vi "Controle_Manip_Main_GUI_Backup2.vi"() -> ()   [LabVIEW 2019] (continued)
                      }
                    }
                    n2428 = local read "ourDLL"() -> (w2916:path)
                    n2429 = call "ANC_MoveAbs.vi"("Att DeviceHandle"=w2915, "ourDLL"=w2916, "axis"=w2918, "Target pos"=w2919, "Att Error"=w2914) -> ("deviceHandle out"=w2913:u64, "Out Position [µm | m°]"=→"Out Position [µm | m°]":dbl, "error out"=w2912:errorcluster)  [unwired: 1 in]
                    n2430 = local write "Att DeviceHandle"(w2913) -> ()
                    n2431 = local write "Att Error"(w2912) -> ()
                  }
                }
              }
              frame #1 {
                n2432 = property on="Att Read Pos" class="Bool (strict)"("Val(Sgnl)"=TRUE ("Value (Signaling)")) -> ()  [unwired: 2 in, 2 out]
              }
            }
          }
          event "Att Read Pos": Value Change {
            n2433 = event-data() -> ()  [unwired: 1 in, 6 out]
            n2434 = flat-sequence {
              frame #0 {
                w2929 = u8 2 items=["1", "2", "3"] ("axis")
                w2930 = u8 1 items=["1", "2", "3"] ("axis")
                w2931 = u8 0 items=["1", "2", "3"] ("axis")
                n2435 = local read "Att DeviceHandle"() -> (w2943:u64)
                n2436 = local read "Att Error"() -> (w2942:errorcluster)
                n2437 = local read "ourDLL"() -> (w2937:path)
                n2438 = call "ANC350v4_GetPosition.vi"("deviceHandle"=w2943, "Path to *.DLL"=w2937, "axis"=w2931, "error in"=w2942) -> ("deviceHandle"=w2941:u64, "Position [µm | m°]"=w2936:dbl, "error ANC350v4_getPosition"=w2940:errorcluster)  [unwired: 8 in, 1 out]
                n2439 = call "ANC350v4_GetPosition.vi"("deviceHandle"=w2941, "Path to *.DLL"=w2937, "axis"=w2930, "error in"=w2940) -> ("deviceHandle"=w2939:u64, "Position [µm | m°]"=w2935:dbl, "error ANC350v4_getPosition"=w2938:errorcluster)  [unwired: 8 in, 1 out]
                n2440 = local write "Att Pos Y"(w2936) -> ()
                n2441 = local write "Att Pos X"(w2935) -> ()
                n2442 = call "ANC350v4_GetPosition.vi"("deviceHandle"=w2939, "Path to *.DLL"=w2937, "axis"=w2929, "error in"=w2938) -> ("deviceHandle"=w2933:u64, "Position [µm | m°]"=w2934:dbl, "error ANC350v4_getPosition"=w2932:errorcluster)  [unwired: 8 in, 1 out]
                n2443 = local write "Att DeviceHandle"(w2933) -> ()
                n2444 = local write "Att Pos Z"(w2934) -> ()
                n2445 = local write "Att Error"(w2932) -> ()
              }
              frame #1 {
                n2446 = local write "Att Read Pos"(FALSE ("Att Read Pos")) -> ()
              }
            }
          }
          event "Att Track Target": Value Change {
            n2447 = event-data() -> ("NewVal"=w2945:bool)  [unwired: 1 in, 5 out]
            n2448 = case shown="False" w2945 {
              frame False {
                w2956 = u8 2 items=["1", "2", "3"] ("axis")
                w2957 = u8 1 items=["1", "2", "3"] ("axis")
                w2962 = u8 0 items=["1", "2", "3"] ("axis")
                n2449 = local read "Att DeviceHandle"() -> (w2950:u64)
                n2450 = local read "Att Error"() -> (w2949:errorcluster)
                n2451 = local read "ourDLL"() -> (w2946:path)
                n2452 = call "ANC350v4_StartAutoMove.vi"("deviceHandle"=w2950, "Path to *.DLL"=w2946, "axis"=w2962, "Enable | Disable"=FALSE, "Relative | Absolute"=TRUE, "error in"=w2949) -> ("deviceHandle out"=w2961:u64, "error ANC350v4_StartAutoMove"=w2960:errorcluster)  [unwired: 7 in, 1 out]
                n2453 = call "ANC350v4_StartAutoMove.vi"("deviceHandle"=w2961, "Path to *.DLL"=w2946, "axis"=w2957, "Enable | Disable"=FALSE, "Relative | Absolute"=TRUE, "error in"=w2960) -> ("deviceHandle out"=w2959:u64, "error ANC350v4_StartAutoMove"=w2958:errorcluster)  [unwired: 7 in, 1 out]
                n2454 = call "ANC350v4_StartAutoMove.vi"("deviceHandle"=w2959, "Path to *.DLL"=w2946, "axis"=w2956, "Enable | Disable"=FALSE, "Relative | Absolute"=TRUE, "error in"=w2958) -> ("deviceHandle out"=w2948:u64, "error ANC350v4_StartAutoMove"=w2947:errorcluster)  [unwired: 7 in, 1 out]
                n2455 = local write "Att DeviceHandle"(w2948) -> ()
                n2456 = local write "Att Error"(w2947) -> ()
              }
              frame True {
              }
            }
          }
          event "Att Up", "Att Down", "Att Left", "Att Right", "Att Backward", "Att Forward": Value Change {
            n2457 = event-data() -> ("CtlRef"=w2965:refnum<vi>, "NewVal"=w2966:bool)  [unwired: 1 in, 4 out]
            n2458 = local read "Voltage Output?"() -> (w2964:bool)
            n2459 = case shown="True" w2964 {
              tunnel: w2966 -> [_ w2969]
              tunnel: w2965 -> [_ w2968]
              frame False {
              }
              frame True {
                n2460 = local read "Att DeviceHandle"() -> (w2974:u64)
                n2461 = local read "ourDLL"() -> (w2971:path)
                n2462 = local read "Att Error"() -> (w2973:errorcluster)
                n2463 = local read "Att Mode"() -> (w2975:enum16{"Single Step", "Continuous", "Automatic"})
                n2464 = property class="Bool (strict)"(reference=w2968) -> ("Label.Text"=w2972:string)  [unwired: 1 in, 2 out]
                n2465 = case shown="\"Automatic\"" w2975 {
                  tunnel: w2974 -> [w2979 w3017 w3064]
                  tunnel: w2973 -> [w2980 w3018 w3063]
                  tunnel: w2972 -> [w2978 w3021 w3045]
                  tunnel: w2971 -> [w2984 w3014 w3056]
                  tunnel: [w2983 w3024 w3068] -> w2970
                  tunnel: [w2982 w3023 w3067] -> w2967
                  tunnel: w2969 -> [_ w3020 _]
                  tunnel: w2968 -> [_ _ w3048]
                  frame "Single Step", Default {
                    n2466 = case shown="\"Att Up\"" w2978 {
                      tunnel: [FALSE ("direction [t=bwd | f=fwd]") TRUE FALSE ("direction [t=bwd | f=fwd]") TRUE ("direction [t=bwd | f=fwd]") FALSE ("direction [t=bwd | f=fwd]") TRUE ("direction [t=bwd | f=fwd]")] -> w2987
                      tunnel: [w3000 w3002 w3005 w3006 w3009 w3010] -> w2981
                      frame "Att Forward" {
                        w3000 = u8 2 items=["1", "2", "3"] ("axis")
                      }
                      frame "Att Backward" {
                        w3002 = u8 2 items=["1", "2", "3"] ("axis")
                      }
                      frame "Att Up" {
                        w3005 = u8 0 items=["1", "2", "3"] ("axis")
                      }
                      frame "Att Down", Default {
                        w3006 = u8 0 items=["1", "2", "3"] ("axis")
                      }
                      frame "Att Left" {
                        w3009 = u8 1 items=["1", "2", "3"] ("axis")
                      }
                      frame "Att Right" {
                        w3010 = u8 1 items=["1", "2", "3"] ("axis")
                      }
                    }
                    n2467 = call "ANC350v4_SingleStep.vi"("deviceHandle"=w2979, "Path to *.DLL"=w2984, "axis"=w2981, "direction [t=bwd | f=fwd]"=w2987, "error in"=w2980) -> ("deviceHandle"=w2985:u64, "error ANC350v4_singleStep"=w2986:errorcluster)  [unwired: 8 in, 1 out]
                    n2468 = call "ANC350v4_GetPosition.vi"("deviceHandle"=w2985, "Path to *.DLL"=w2984, "axis"=w2981, "error in"=w2986) -> ("deviceHandle"=w2983:u64, "Position [µm | m°]"=w2977:dbl, "error ANC350v4_getPosition"=w2982:errorcluster)  [unwired: 8 in, 1 out]
                    n2469 = case shown="\"Att Backward\"" w2978 {
                      tunnel: w2977 -> [w2989 w2991 w2993 w2995 w2997 _ w2999]
                      tunnel: FALSE -> [w2988 w2990 w2992 w2994 w2996 _ w2998]
                      frame "Att Right" {
                        n2470 = local write "Att Right"(w2988) -> ()
                        n2471 = local write "Att Pos X"(w2989) -> ()
                      }
                      frame "Att Left" {
                        n2472 = local write "Att Left"(w2990) -> ()
                        n2473 = local write "Att Pos X"(w2991) -> ()
                      }
                      frame "Att Up" {
                        n2474 = local write "Att Up"(w2992) -> ()
                        n2475 = local write "Att Pos Y"(w2993) -> ()
                      }
                      frame "Att Down" {
                        n2476 = local write "Att Down"(w2994) -> ()
                        n2477 = local write "Att Pos Y"(w2995) -> ()
                      }
                      frame "Att Forward" {
                        n2478 = local write "Att Forward"(w2996) -> ()
                        n2479 = local write "Att Pos Z"(w2997) -> ()
                      }
                      frame "False", Default {
                      }
                      frame "Att Backward" {
                        n2480 = local write "Att Backward"(w2998) -> ()
                        n2481 = local write "Att Pos Z"(w2999) -> ()
                      }
                    }
                  }
                  frame "Continuous" {
                    n2482 = case shown="False" w3020 {
                      tunnel: [FALSE TRUE] -> w3015
                      frame False {
                      }
                      frame True {
                      }
                    }
                    n2483 = case shown="\"Att Left\"" w3021 {
                      tunnel: [FALSE ("direction [t=bwd | f=fwd]") TRUE FALSE ("direction [t=bwd | f=fwd]") TRUE ("direction [t=bwd | f=fwd]") FALSE ("direction [t=bwd | f=fwd]") TRUE ("direction [t=bwd | f=fwd]")] -> w3019
                      tunnel: [w3033 w3035 w3038 w3039 w3042 w3043] -> w3016
                      frame "Att Forward" {
                        w3033 = u8 2 items=["1", "2", "3"] ("axis")
                      }
                      frame "Att Backward" {
                        w3035 = u8 2 items=["1", "2", "3"] ("axis")
                      }
                      frame "Att Up" {
                        w3038 = u8 0 items=["1", "2", "3"] ("axis")
                      }
                      frame "Att Down", Default {
                        w3039 = u8 0 items=["1", "2", "3"] ("axis")
                      }
                      frame "Att Left" {
                        w3042 = u8 1 items=["1", "2", "3"] ("axis")
                      }
                      frame "Att Right" {
                        w3043 = u8 1 items=["1", "2", "3"] ("axis")
                      }
                    }
                    n2484 = call "ANC350v4_StartContinousMove.vi"("deviceHandle"=w3017, "Path to *.DLL"=w3014, "axis"=w3016, "start | stop"=w3015, "direction [t=bwd | f=fwd]"=w3019, "error in"=w3018) -> ("deviceHandle"=w3012:u64, "error ANC350v4_startContinousMove"=w3013:errorcluster)  [unwired: 7 in, 1 out]
                    n2485 = call "ANC350v4_GetPosition.vi"("deviceHandle"=w3012, "Path to *.DLL"=w3014, "axis"=w3016, "error in"=w3013) -> ("deviceHandle"=w3024:u64, "Position [µm | m°]"=w3022:dbl, "error ANC350v4_getPosition"=w3023:errorcluster)  [unwired: 8 in, 1 out]
                    n2486 = case shown="\"Att Right\"" w3021 {
                      tunnel: w3022 -> [_ w3027 w3028 w3029 w3030 w3031 w3032]
                      frame "False", Default {
                      }
                      frame "Att Right" {
                        n2487 = local write "Att Pos X"(w3027) -> ()
                      }
                      frame "Att Left" {
                        n2488 = local write "Att Pos X"(w3028) -> ()
                      }
                      frame "Att Up" {
                        n2489 = local write "Att Pos Y"(w3029) -> ()
                      }
                      frame "Att Down" {
                        n2490 = local write "Att Pos Y"(w3030) -> ()
                      }
                      frame "Att Forward" {
                        n2491 = local write "Att Pos Z"(w3031) -> ()
                      }
                      frame "Att Backward" {
                        n2492 = local write "Att Pos Z"(w3032) -> ()
                      }
                    }
                  }
                  frame "Automatic" {
                    n2493 = local read "Att AutoStep"() -> (w3046:dbl)
                    n2494 = case shown="\"Att Right\"" w3045 {
                      tunnel: [w3110 w3113 w3115 w3118 w3120 w3123] -> w3057
                      tunnel: [w3109 w3111 w3114 w3117 w3119 w3121] -> w3047
                      tunnel: w3046 -> [w3109 w3112 w3114 w3116 w3119 w3122]
                      frame "Att Forward" {
                        w3110 = u8 2 items=["1", "2", "3"] ("axis")
                      }
                      frame "Att Backward" {
                        w3113 = u8 2 items=["1", "2", "3"] ("axis")
                        n2495 = Negate(x=w3112) -> (-x=w3111:dbl)
                      }
                      frame "Att Up" {
                        w3115 = u8 0 items=["1", "2", "3"] ("axis")
                      }
                      frame "Att Down", Default {
                        w3118 = u8 0 items=["1", "2", "3"] ("axis")
                        n2496 = Negate(x=w3116) -> (-x=w3117:dbl)
                      }
                      frame "Att Left" {
                        w3120 = u8 1 items=["1", "2", "3"] ("axis")
                      }
                      frame "Att Right" {
                        w3123 = u8 1 items=["1", "2", "3"] ("axis")
                        n2497 = Negate(x=w3122) -> (-x=w3121:dbl)
                      }
                    }
                    n2498 = call "ANC350v4_SetTarget.vi"("deviceHandle"=w3064, "Path to *.DLL"=w3056, "axis"=w3057, "Target [µm | m°]"=w3047, "error in"=w3063) -> ("deviceHandle"=w3065:u64, "error ANC350v4_setTarget"=w3062:errorcluster)  [unwired: 8 in, 1 out]
                    n2499 = call "ANC350v4_StartAutoMove.vi"("deviceHandle"=w3065, "Path to *.DLL"=w3056, "axis"=w3057, "Enable | Disable"=TRUE, "Relative | Absolute"=TRUE, "error in"=w3062) -> ("deviceHandle out"=w3058:u64, "error ANC350v4_StartAutoMove"=w3059:errorcluster)  [unwired: 7 in, 1 out]
                    n2500 = while {
                      tunnel: w3059 -> [w3102]
                      tunnel: w3058 -> [w3101]
                      tunnel: w3057 -> [w3091]
                      tunnel: w3056 -> [w3090]
                      tunnel: [w3094] -> w3052
                      tunnel: [w3093] -> w3051
                      tunnel: [w3090] -> w3050
                      tunnel: [w3091] -> w3049
                      tunnel: w3045 -> [w3089]
                      stop <- w3098 stop-if-true
                      n2501 = call "ANC350v4_GetAxisStatus.vi"("deviceHandle"=w3101, "Path to *.DLL"=w3090, "axis"=w3091, "error in"=w3102) -> ("deviceHandle"=w3095:u64, "Target"=w3099:bool, "error ANC350v4_getAxisStatus"=w3092:errorcluster)  [unwired: 6 in, 3 out]
                      n2502 = Wait (ms)(milliseconds to wait=u32 250) -> ()  [unwired: 1 out]
                      n2503 = call "ANC350v4_GetPosition.vi"("deviceHandle"=w3095, "Path to *.DLL"=w3090, "axis"=w3091, "error in"=w3092) -> ("deviceHandle"=w3094:u64, "Position [µm | m°]"=w3096:dbl, "error ANC350v4_getPosition"=w3093:errorcluster)  [unwired: 8 in, 1 out]
                      n2504 = case shown="\"Att Down\"" w3089 {
                        tunnel: w3096 -> [_ w3103 w3104 w3105 w3106 w3107 w3108]
                        frame "False", Default {
                        }
                        frame "Att Right" {
                          n2505 = local write "Att Pos X"(w3103) -> ()
                        }
                        frame "Att Left" {
                          n2506 = local write "Att Pos X"(w3104) -> ()
                        }
                        frame "Att Up" {
                          n2507 = local write "Att Pos Y"(w3105) -> ()
                        }
                        frame "Att Down" {
                          n2508 = local write "Att Pos Y"(w3106) -> ()
                        }
                        frame "Att Forward" {
                          n2509 = local write "Att Pos Z"(w3107) -> ()
                        }
                        frame "Att Backward" {
                          n2510 = local write "Att Pos Z"(w3108) -> ()
                        }
                      }
                      n2511 = Or(x=w3099, y="Att Stop Target Wait") -> (x .or. y?=w3098:bool)
                    }
                    n2512 = local read "Att Track Target"() -> (w3053:bool)
                    n2513 = case shown="False" w3053 {
                      tunnel: w3052 -> [w3085 w3088]
                      tunnel: w3051 -> [w3084 w3087]
                      tunnel: [w3082 w3088] -> w3055
                      tunnel: [w3083 w3087] -> w3054
                      tunnel: w3050 -> [w3086 _]
                      tunnel: w3049 -> [w3081 _]
                      frame False {
                        n2514 = call "ANC350v4_StartAutoMove.vi"("deviceHandle"=w3085, "Path to *.DLL"=w3086, "axis"=w3081, "Enable | Disable"=FALSE, "Relative | Absolute"=TRUE, "error in"=w3084) -> ("deviceHandle out"=w3082:u64, "error ANC350v4_StartAutoMove"=w3083:errorcluster)  [unwired: 7 in, 1 out]
                      }
                      frame True {
                      }
                    }
                    n2515 = call "ANC350v4_GetPosition.vi"("deviceHandle"=w3055, "Path to *.DLL"=w3056, "axis"=w3057, "error in"=w3054) -> ("deviceHandle"=w3068:u64, "Position [µm | m°]"=w3066:dbl, "error ANC350v4_getPosition"=w3067:errorcluster)  [unwired: 8 in, 1 out]
                    n2516 = stacked-sequence {
                      tunnel: w3066 -> [w3070 _]
                      tunnel: w3045 -> [w3069 _]
                      tunnel: w3048 -> [_ w3077]
                      frame #0 {
                        n2517 = case shown="\"Att Right\"" w3069 {
                          tunnel: w3070 -> [_ w3071 w3072 w3073 w3074 w3075 w3076]
                          frame "False", Default {
                          }
                          frame "Att Right" {
                            n2518 = local write "Att Pos X"(w3071) -> ()
                          }
                          frame "Att Left" {
                            n2519 = local write "Att Pos X"(w3072) -> ()
                          }
                          frame "Att Up" {
                            n2520 = local write "Att Pos Y"(w3073) -> ()
                          }
                          frame "Att Down" {
                            n2521 = local write "Att Pos Y"(w3074) -> ()
                          }
                          frame "Att Forward" {
                            n2522 = local write "Att Pos Z"(w3075) -> ()
                          }
                          frame "Att Backward" {
                            n2523 = local write "Att Pos Z"(w3076) -> ()
                          }
                        }
                      }
                      frame #1 {
                        n2524 = property class="Bool (strict)"(reference=w3077, "Value"=FALSE) -> ()  [unwired: 1 in, 2 out]
                      }
                    }
                  }
                }
                n2525 = local write "Att DeviceHandle"(w2970) -> ()
                n2526 = local write "Att Error"(w2967) -> ()
              }
            }
          }
          event "Att Wobble Get Pos 1", "Att Wobble Get Pos 2", "Att Wobble": Mouse Down {
            n2527 = event-data() -> ("CtlRef"=w3125:refnum<vi>)  [unwired: 1 in, 7 out]
            n2528 = property class="Bool (strict)"(reference=w3125) -> ("Label.Text"=w3124:string)  [unwired: 1 in, 2 out]
            n2529 = case shown="\"Att Wobble\"" w3124 {
              frame "Att Wobble" {
                n2530 = stacked-sequence {
                  frame #0 {
                    n2531 = local read "Att DeviceHandle"() -> (w3132:u64)
                    n2532 = local read "Att Wobble Start"() -> (w3134:dbl)
                    n2533 = local read "Att Wobble End"() -> (w3133:dbl)
                    n2534 = control-ref of="Att Wobble Stop2"() -> (w3127:refnum<vi>)
                    n2535 = local read "Att Error"() -> (w3131:errorcluster)
                    n2536 = local read "ourDLL"() -> (w3130:path)
                    n2537 = control-ref of="Att Pos Z"() -> (w3126:refnum<vi>)
                    n2538 = call "Att_Wobble.vi"("Att Pos Z"=w3126, "Att Wobble End"=w3133, "Att Wobble Start"=w3134, "Att Error"=w3131, "ourDLL"=w3130, "Att Wobble Stop2 2"=w3127, "Att DeviceHandle"=w3132) -> ("Att Error out"=w3128:errorcluster, "Att DeviceHandle out"=w3129:u64)  [unwired: 1 in]
                    n2539 = local write "Att DeviceHandle"(w3129) -> ()
                    n2540 = local write "Att Error"(w3128) -> ()
                  }
                  frame #1 {
                    w3135 = FALSE ("Att Wobble")
                    n2541 = local write "Att Wobble Stop2"(w3135) -> ()
                    n2542 = local write "Att Wobble"(w3135) -> ()
                  }
                }
              }
              frame "False", Default {
              }
              frame "Att Wobble Get Pos 1" {
                n2543 = property on="Att Pos Z" class="DigNum (strict)"() -> ("Value"=w3136:dbl)  [unwired: 2 in, 2 out]
                n2544 = local write "Att Wobble Start"(w3136) -> ()
              }
              frame "Att Wobble Get Pos 2" {
                n2545 = property on="Att Pos Z" class="DigNum (strict)"() -> ("Value"=w3137:dbl)  [unwired: 2 in, 2 out]
                n2546 = local write "Att Wobble End"(w3137) -> ()
              }
            }
          }
          event "Auto< ?": Value Change {
            n2547 = event-data() -> ("NewVal"=w3138:bool)  [unwired: 1 in, 5 out]
            n2548 = case shown="True" w3138 {
              frame False {
                w3139 = TRUE ("Visible")
                n2549 = property on="Save Spectrum N" class="Bool (strict)"("Visible"=w3139) -> ()  [unwired: 2 in, 2 out]
                n2550 = property on="Save XY Map" class="Bool (strict)"("Visible"=w3139) -> ()  [unwired: 2 in, 2 out]
                n2551 = property on="Save Spectrum" class="Bool (strict)"("Visible"=w3139) -> ()  [unwired: 2 in, 2 out]
                n2552 = property on="Save PLE" class="Bool (strict)"("Visible"=w3139) -> ()  [unwired: 2 in, 2 out]
                n2553 = property on="Save fPow" class="Bool (strict)"("Visible"=w3139) -> ()  [unwired: 2 in, 2 out]
                n2554 = property on="Save Custom Diode Spectrum" class="Bool (strict)"("Visible"=w3139) -> ()  [unwired: 2 in, 2 out]
                n2555 = property on="Save Michelson" class="Bool (strict)"("Visible"=w3139) -> ()  [unwired: 2 in, 2 out]
                n2556 = property on="Save Polarisation" class="Bool (strict)"("Visible"=w3139) -> ()  [unwired: 2 in, 2 out]
                n2557 = property on="Save Contrast" class="Bool (strict)"("Visible"=w3139) -> ()  [unwired: 2 in, 2 out]
              }
              frame True {
                w3140 = FALSE ("Visible")
                n2558 = property on="Save Spectrum N" class="Bool (strict)"("Visible"=w3140) -> ()  [unwired: 2 in, 2 out]
                n2559 = property on="Save XY Map" class="Bool (strict)"("Visible"=w3140) -> ()  [unwired: 2 in, 2 out]
                n2560 = property on="Save Spectrum" class="Bool (strict)"("Visible"=w3140) -> ()  [unwired: 2 in, 2 out]
                n2561 = property on="Save PLE" class="Bool (strict)"("Visible"=w3140) -> ()  [unwired: 2 in, 2 out]
                n2562 = property on="Save fPow" class="Bool (strict)"("Visible"=w3140) -> ()  [unwired: 2 in, 2 out]
                n2563 = property on="Save Polarisation" class="Bool (strict)"("Visible"=w3140) -> ()  [unwired: 2 in, 2 out]
                n2564 = property on="Save Michelson" class="Bool (strict)"("Visible"=w3140) -> ()  [unwired: 2 in, 2 out]
                n2565 = property on="Save Contrast" class="Bool (strict)"("Visible"=w3140) -> ()  [unwired: 2 in, 2 out]
                n2566 = property on="Save Custom Diode Spectrum" class="Bool (strict)"("Visible"=w3140) -> ()  [unwired: 2 in, 2 out]
              }
            }
          }
          event "Background substract": Value Change {
            n2567 = event-data() -> ("NewVal"=w3141:enum16{"None", "Shutter"})  [unwired: 1 in, 5 out]
            n2568 = case shown="\"Shutter\"" w3141 {
              frame "None", Default {
              }
              frame "Shutter" {
                n2569 = stacked-sequence {
                  tunnel: [_ _ w3191] -> w3142
                  frame #0 {
                    n2570 = local read "Log file"() -> (w3176:string)
                    n2571 = property on="CCD 1D Spectrum Main" class="XYGraph (strict)"("YScale.Offset"=0.0 ("Y Scale.Offset and Multiplier:Offset")) -> ()  [unwired: 2 in, 2 out]
                    n2572 = call "Write2LogFile.vi"("Add to log file"="Acquiring background", "Log file before"=w3176, "Checkbox"=FALSE) -> ("Log file after"=w3175:string)
                    n2573 = local write "Log file"(w3175) -> ()
                  }
                  frame #1 {
                    # "make sure shutter is closed"
                    n2574 = local read "KCube Shutter On?"() -> (w3177:bool)
                    n2575 = control-ref of="Shutter Ctrls"() -> (w3181:refnum<vi>)
                    n2576 = property class="Ring (strict)"(reference=w3181) -> ("Value"=w3180:u16)  [unwired: 1 in, 2 out]
                    n2577 = control-ref of="KCube Shutter Device Reference"() -> (w3182:refnum<vi>)
                    n2578 = Equal?(x=w3180, y=u16 0) -> (x = y?=w3178:bool)
                    n2579 = case shown="False" w3178 {
                      tunnel: w3182 -> [w3185 _]
                      tunnel: w3181 -> [w3184 _]
                      tunnel: w3177 -> [w3183 _]
                      frame False {
                        n2580 = call "Shutter.vi"("KCube Shutter Device Reference 2"=w3185, "Shutter Ctrls 2"=w3184, "Shutter on?"=w3183) -> ()
                      }
                      frame True {
                      }
                    }
                  }
                  frame #2 {
                    # "acquire"
                    n2581 = local read "LightField Automation error out"() -> (w3189:errorcluster)
                    n2582 = local read "LightField Automation out"() -> (w3190:refnum<class "LightField Automation.lvclass">)
                    n2583 = local read "Accumulations"() -> (w3186:dbl)
                    n2584 = call "LFA_Capture.vi"("error in (no error)"=w3189, "Frames"=w3186, "LightField Automation in"=w3190) -> ("error out"=w3188:errorcluster, "Data"=w3191:T26, "LightField Automation out"=w3187:refnum<class "LightField Automation.lvclass">)  [unwired: 6 in]
                    n2585 = local write "LightField Automation error out"(w3188) -> ()
                    n2586 = local write "LightField Automation out"(w3187) -> ()
                  }
                }
                n2587 = local read "Acq Mode"() -> (w3143:T3)
                n2588 = case shown="\"Spectrum\", Default" w3143 {
                  selector: w3143 -> [w3144 w3162]
                  tunnel: w3142 -> [w3145 w3163]
                  frame "Spectrum", Default {
                    n2589 = stacked-sequence {
                      tunnel: w3145 -> [_ w3156 _ _]
                      tunnel: w3144 -> [_ w3154 _ _]
                      frame #0 {
                        n2590 = property on="CCD 2D Image Main" class="IntGraph (strict)"("Visible"=FALSE) -> ()  [unwired: 2 in, 2 out]
                        n2591 = property on="CCD 1D Spectrum Main" class="XYGraph (strict)"("Visible"=TRUE) -> ()  [unwired: 2 in, 2 out]
                      }
                      frame #1 {
                        n2592 = local read "CCD ROI"() -> (w3149:T20)
                        n2593 = local read "Wavelength calibration"() -> (w3153:dbl[])
                        n2594 = Divide(x=1239.842, y=w3153) -> (x/y=w3151:dbl[])
                        n2595 = call "PrepareData4Graph.vi"("Wavelength nm"=w3151, "DataLF"=w3156, "CCD ROI"=w3149, "AcqMode"=w3154, "Data type"=T30."Spectre") -> ("Spectrum"=w3155:cluster{"Array 2":dbl[], "Array":dbl[]}, "PLInt out"=w3148:dbl[])  [unwired: 2 in, 2 out]
                        n2596 = local write "CCD 1D Spectrum Main"(w3155) -> ()
                        n2597 = local write "BackgroundSpec"(w3148) -> ()
                      }
                      frame #2 {
                        n2598 = local read "BackgroundSpec"() -> (w3157:dbl[])
                        n2599 = call-poly <vilib>:"Mean.vi"("X"=w3157) -> ("mean"=w3159:dbl)  [unwired: 1 out]
                        n2600 = Negate(x=w3159) -> (-x=w3158:dbl)
                        n2601 = property on="CCD 1D Spectrum Main" class="XYGraph (strict)"("YScale.Offset"=w3158) -> ()  [unwired: 2 in, 2 out]
                      }
                      frame #3 {
                        n2602 = local write "Background taken?"(TRUE ("Background taken?")) -> ()
                        n2603 = property on="Background substract" class="Enum (strict)"("Value"=enum16{"None", "Shutter"}."None" ("Background substract")) -> ()  [unwired: 2 in, 2 out]
                      }
                    }
                  }
                  frame "Image" {
                    n2604 = stacked-sequence {
                      tunnel: w3163 -> [_ w3171]
                      tunnel: w3162 -> [_ w3169]
                      frame #0 {
                        n2605 = property on="CCD 1D Spectrum Main" class="XYGraph (strict)"("Visible"=FALSE) -> ()  [unwired: 2 in, 2 out]
                        n2606 = property on="CCD 2D Image Main" class="IntGraph (strict)"("Visible"=TRUE) -> ()  [unwired: 2 in, 2 out]
                      }
                      frame #1 {
                        n2607 = local read "Wavelength calibration"() -> (w3170:dbl[])
                        n2608 = local read "CCD ROI"() -> (w3166:T20)
                        n2609 = call "PrepareData4Graph.vi"("Wavelength nm"=w3170, "DataLF"=w3171, "CCD ROI"=w3166, "AcqMode"=w3169, "Data type"=T30."Spectre") -> ("Intensity Graph"=w3168:dbl[][])  [unwired: 2 in, 3 out]
                        n2610 = local write "CCD 2D Image Main"(w3168) -> ()
                      }
                    }
                  }
                }
              }
            }
          }
          event "CCD 1D Spectrum Main  Cursor2WL 1 Mono 1", "CCD 1D Spectrum Main  Cursor2WL 2 Mono 1", "CCD 1D Spectrum Main  Cursor2WL 1 Mono 2", "CCD 1D Spectrum Main  Cursor2WL 2 Mono 2": Mouse Down {
            n2611 = event-data() -> ("CtlRef"=w3193:refnum<vi>)  [unwired: 1 in, 7 out]
            n2612 = property class="Bool (strict)"(reference=w3193) -> ("Label.Text"=w3192:string)  [unwired: 1 in, 2 out]
            n2613 = case shown="Default" w3192 {
              frame "CCD 1D Spectrum Main  Cursor2WL 1 Mono 1" {
                n2614 = local read "CCD 1D Spectrum Main Cursor 1 nm"() -> (w3194:dbl)
                n2615 = property on="Center Wavelength (nm)" class="DigNum (strict)"("Val(Sgnl)"=w3194) -> ()  [unwired: 2 in, 2 out]
              }
              frame "CCD 1D Spectrum Main  Cursor2WL 1 Mono 2" {
                n2616 = local read "CCD 1D Spectrum Main Cursor 1 nm"() -> (w3195:dbl)
                n2617 = property on="Mono2 Wavelength (nm)" class="DigNum (strict)"("Val(Sgnl)"=w3195) -> ()  [unwired: 2 in, 2 out]
              }
              frame "CCD 1D Spectrum Main  Cursor2WL 2 Mono 2" {
                n2618 = local read "CCD 1D Spectrum Main Cursor 2 nm"() -> (w3196:dbl)
                n2619 = property on="Mono2 Wavelength (nm)" class="DigNum (strict)"("Val(Sgnl)"=w3196) -> ()  [unwired: 2 in, 2 out]
              }
              frame "CCD 1D Spectrum Main  Cursor2WL 2 Mono 1" {
                n2620 = local read "CCD 1D Spectrum Main Cursor 2 nm"() -> (w3197:dbl)
                n2621 = property on="Center Wavelength (nm)" class="DigNum (strict)"("Val(Sgnl)"=w3197) -> ()  [unwired: 2 in, 2 out]
              }
              frame Default {
              }
            }
          }
          event "CCD 1D Spectrum Main", "Contrast Oscillations", "Contrast 1D Spectrum": Cursor Release {
            n2622 = event-data() -> ("CtlRef"=w3201:refnum<vi>, "CursRef"=w3199:refnum<vi>)  [unwired: 1 in, 7 out]
            n2623 = property class="XYGraph (strict)"(reference=w3201) -> ("Label.Text"=w3200:string)  [unwired: 1 in, 2 out]
            n2624 = property class="Curs"(reference=w3199) -> ("Cursor Name"=w3198:string)  [unwired: 1 in, 2 out]
            n2625 = case shown="\"Contrast 1D Spectrum\"" w3200 {
              tunnel: w3198 -> [w3202 _ _ _]
              frame "Contrast Oscillations" {
                n2626 = case shown="\"ContPos\"" w3202 {
                  frame "False", Default {
                  }
                  frame "ContPos" {
                    n2627 = local read "Cursor controls"() -> (w3203:bool)
                    n2628 = case shown="True" w3203 {
                      frame False {
                      }
                      frame True {
                        n2629 = property on="Contrast Oscillations" class="XYGraph (strict)"("Active Cursor"=u32 2) -> ("Cursor.Cursor X"=w3204:dbl)  [unwired: 2 in, 2 out]
                        n2630 = Number To Decimal String(number=w3204) -> (decimal integer string=w3206:string)  [unwired: 1 in]
                        n2631 = property on="Contrast 1D Spectrum from Cursors" class="XYGraph (strict)"("Caption.Text"=w3206) -> ()  [unwired: 2 in, 2 out]
                      }
                    }
                  }
                  frame "ContInt1" {
                    n2632 = property on="Contrast Oscillations" class="XYGraph (strict)"("Active Cursor"=u32 0, "Active Cursor"=u32 1) -> ("Cursor.Cursor Y"=w3209:dbl, "Cursor.Cursor Y"=w3208:dbl)  [unwired: 2 in, 2 out]
                    n2633 = call "Contrast.vi"("Y2"=w3208, "Y1"=w3209) -> ("(max(Y1,Y2) - min(Y1,Y2)) / (Y1 + Y2)"=w3207:dbl)
                    n2634 = local write "Contrast"(w3207) -> ()
                  }
                  frame "ContInt2" {
                    n2635 = property on="Contrast Oscillations" class="XYGraph (strict)"("Active Cursor"=u32 0, "Active Cursor"=u32 1) -> ("Cursor.Cursor Y"=w3214:dbl, "Cursor.Cursor Y"=w3213:dbl)  [unwired: 2 in, 2 out]
                    n2636 = call "Contrast.vi"("Y2"=w3213, "Y1"=w3214) -> ("(max(Y1,Y2) - min(Y1,Y2)) / (Y1 + Y2)"=w3212:dbl)
                    n2637 = local write "Contrast"(w3212) -> ()
                  }
                }
              }
              frame "Contrast 1D Spectrum" {
                n2638 = case shown="True" "Cursor controls" {
                  frame False {
                  }
                  frame True {
                    n2639 = property on="Contrast 1D Spectrum" class="XYGraph (strict)"("Active Cursor"=u32 0, "Active Cursor"=u32 1) -> ("Cursor.Cursor X"=w3225:dbl, "Cursor.Cursor X"=w3224:dbl)  [unwired: 2 in, 2 out]
                    n2640 = local read "Wavelength calibration"() -> (w3230:dbl[])
                    n2641 = local read "Contrast Array Out"() -> (w3226:dbl[][])
                    n2642 = Divide(x=1239.842, y=w3230) -> (x/y=w3227:dbl[])
                    n2643 = call "Cursors4Contrast_v2.vi"("Cursor 2"=w3224, "Cursor 1"=w3225, "Spectres vs PZA"=w3226, "Energy"=w3227) -> ("Contrast of ROI vs PZC"=w3223:dbl[], "Spectra ROI"=w3220:dbl[][], "Energy ROI"=w3222:dbl[])
                    n2644 = Index Array(array=w3220, index (row)=0) -> (element=w3218:dbl[])  [unwired: 1 in]
                    n2645 = local read "PZA12 Positions"() -> (w3229:dbl[])
                    n2646 = Bundle("Energy ROI"=w3222, "Spectra ROI"=w3218) -> (w3221:cluster{"Energy ROI":dbl[], "Spectra ROI":dbl[]})  [unwired: 1 in]
                    n2647 = property on="Contrast 1D Spectrum from Cursors" class="XYGraph (strict)"("Value"=w3221) -> ()  [unwired: 2 in, 2 out]
                    n2648 = Bundle("PZA12 Positions"=w3229, "Contrast of ROI vs PZC"=w3223) -> (w3228:T38)  [unwired: 1 in]
                    n2649 = property on="Contrast Oscillations" class="XYGraph (strict)"("Value"=w3228) -> ()  [unwired: 2 in, 2 out]
                  }
                }
              }
              frame Default {
              }
              frame "CCD 1D Spectrum Main" {
                n2650 = stacked-sequence {
                  seq-local: [w3235 _] -> [_ w3243]
                  seq-local: [w3234 _] -> [_ w3242]
                  frame #0 {
                    n2651 = property on="CCD 1D Spectrum Main" class="XYGraph (strict)"("Active Cursor"=u32 0, "Active Cursor"=u32 1) -> ("Cursor.Cursor X"=w3235:dbl, "Cursor.Cursor X"=w3234:dbl)  [unwired: 2 in, 2 out]
                    n2652 = local write "CCD 1D Spectrum Main Cursor"(w3235) -> ()
                    n2653 = local write "CCD 1D Spectrum Main Cursor 2"(w3234) -> ()
                  }
                  frame #1 {
                    n2654 = call "Cursors2Freq.vi"("Cursor 1 eV"=w3243, "Cursor 2 eV"=w3242) -> ("Cursor dE"=w3241:dbl, "Cursor 1 nm"=w3240:dbl, "Cursor 2 nm"=w3239:dbl, "Cursor dnm"=w3238:dbl)
                    n2655 = local write "CCD 1D Spectrum Main deltaE"(w3241) -> ()
                    n2656 = local write "CCD 1D Spectrum Main Cursor 1 nm"(w3240) -> ()
                    n2657 = local write "CCD 1D Spectrum Main Cursor 2 nm"(w3239) -> ()
                    n2658 = Multiply(x=w3238, y=1e-09) -> (x*y=w3244:dbl)
                    n2659 = local write "CCD 1D Spectrum Main deltanm"(w3244) -> ()
                  }
                }
              }
            }
          }
          event "CCD 1D Spectrum Main", "Polarisation 1D Spectrum", "CCD 1D Spectrum XY Map": Scale Range Change {
            n2660 = event-data() -> ("CtlRef"=w3246:refnum<vi>, "ScaleRef"=w3249:refnum<vi>, "NewRange"=w3247:T39)  [unwired: 1 in, 5 out]
            n2661 = property class="GrphScl"(reference=w3249) -> ("NameLbl.Text"=w3248:string)  [unwired: 1 in, 2 out]
            n2662 = case shown="\"Energy (eV)\"" w3248 {
              tunnel: w3246 -> [w3254 _]
              tunnel: w3247 -> [w3252 _]
              frame "Energy (eV)" {
                w3253 = 1239.842
                n2663 = property class="XYGraph (strict)"(reference=w3254) -> ("Label.Text"=w3257:string)  [unwired: 1 in, 2 out]
                n2664 = Unbundle By Name(w3252) -> ("Minimum"=w3251:dbl, "Maximum"=w3250:dbl)
                n2665 = Divide(x=w3253, y=w3251) -> (x/y=w3255:dbl)
                n2666 = Divide(x=w3253, y=w3250) -> (x/y=w3256:dbl)
                n2667 = case shown="\"CCD 1D Spectrum Main\", Default" w3257 {
                  tunnel: w3255 -> [w3262 w3288 w3294]
                  tunnel: w3256 -> [w3263 w3287 w3295]
                  tunnel: w3251 -> [w3258 w3284 _]
                  tunnel: w3250 -> [w3259 w3283 _]
                  frame "CCD 1D Spectrum Main", Default {
                    n2668 = disable-structure shown="Disabled" {
                      disable-tunnel: w3259 -> [w3265 _]
                      disable-tunnel: w3258 -> [w3264 _]
                      frame Disabled {
                        n2669 = property on="CCD 1D Spectrum Main" class="XYGraph (strict)"("Active Cursor"=1 ("Cursor.Cursor Index")) -> ("Cursor.Cursor X"=w3268:dbl)  [unwired: 2 in, 2 out]
                        n2670 = property on="CCD 1D Spectrum Main" class="XYGraph (strict)"("Active Cursor"=0 ("Cursor.Cursor Index")) -> ("Cursor.Cursor X"=w3270:dbl)  [unwired: 2 in, 2 out]
                        n2671 = In Range and Coerce(upper limit=w3265, x=w3270, lower limit=w3264) -> (In Range?=w3271:bool)  [unwired: 1 out]
                        n2672 = In Range and Coerce(upper limit=w3265, x=w3268, lower limit=w3264) -> (In Range?=w3267:bool)  [unwired: 1 out]
                        n2673 = Not(x=w3271) -> (.not. x?=w3272:bool)
                        n2674 = Not(x=w3267) -> (.not. x?=w3266:bool)
                        n2675 = case shown="True" w3272 {
                          tunnel: w3264 -> [_ w3276]
                          frame False {
                          }
                          frame True {
                            n2676 = property on="CCD 1D Spectrum Main" class="XYGraph (strict)"("Active Cursor"=0 ("Cursor.Cursor Index"), "Cursor.Cursor X"=w3276) -> ()  [unwired: 2 in, 2 out]
                          }
                        }
                        n2677 = case shown="True" w3266 {
                          tunnel: w3265 -> [_ w3274]
                          frame False {
                          }
                          frame True {
                            n2678 = property on="CCD 1D Spectrum Main" class="XYGraph (strict)"("Active Cursor"=1 ("Cursor.Cursor Index"), "Cursor.Cursor X"=w3274) -> ()  [unwired: 2 in, 2 out]
                          }
                        }
                      }
                      frame Enabled {
                      }
                    }
                    n2679 = property on="CCD 1D Spectrum Main Energy Scale" class="XYGraph (strict)"("XScale.Maximum"=w3262, "XScale.Minimum"=w3263, "XScale.UniformMarker"=TRUE ("X Scale.Uniform Marker Spacing?")) -> ()  [unwired: 2 in, 2 out]
                    n2680 = for {
                      N: 2 -> [_]
                      tunnel: w3259 -> [w3282]
                      tunnel: w3258 -> [w3281]
                      i -> [w3278]
                      # "coerce both cursors to new range"
                      n2681 = property on="CCD 1D Spectrum Main" class="XYGraph (strict)"("Active Cursor"=w3278) -> ("Cursor.Cursor X"=w3280:dbl)  [unwired: 2 in, 2 out]
                      n2682 = In Range and Coerce(upper limit=w3282, x=w3280, lower limit=w3281) -> (coerced(x)=w3279:dbl)  [unwired: 1 out]
                      n2683 = property on="CCD 1D Spectrum Main" class="XYGraph (strict)"("Active Cursor"=w3278, "Cursor.Cursor X"=w3279) -> ()  [unwired: 2 in, 2 out]
                    }
                  }
                  frame "CCD 1D Spectrum XY Map" {
                    n2684 = for {
                      N: 2 -> [_]
                      tunnel: w3284 -> [w3293]
                      tunnel: w3283 -> [w3292]
                      i -> [w3289]
                      # "coerce both cursors to new range"
                      n2685 = property on="CCD 1D Spectrum XY Map" class="XYGraph (strict)"("Active Cursor"=w3289) -> ("Cursor.Cursor X"=w3291:dbl)  [unwired: 2 in, 2 out]
                      n2686 = In Range and Coerce(upper limit=w3292, x=w3291, lower limit=w3293) -> (coerced(x)=w3290:dbl)  [unwired: 1 out]
                      n2687 = property on="CCD 1D Spectrum XY Map" class="XYGraph (strict)"("Active Cursor"=w3289, "Cursor.Cursor X"=w3290) -> ()  [unwired: 2 in, 2 out]
                    }
                    n2688 = property on="CCD 1D XY Map Spectrum Main Energy Scale" class="XYGraph (strict)"("XScale.Minimum"=w3287, "XScale.Maximum"=w3288, "XScale.UniformMarker"=TRUE ("X Scale.Uniform Marker Spacing?")) -> ()  [unwired: 2 in, 2 out]
                  }
                  frame "Polarisation 1D Spectrum" {
                    n2689 = property on="Polarisation 1D Spectrum Energy Scale" class="XYGraph (strict)"("XScale.Maximum"=w3294, "XScale.Minimum"=w3295) -> ()  [unwired: 2 in, 2 out]
                    n2690 = property on="CCD 1D XY Map Spectrum Main Energy Scale" class="XYGraph (strict)"("XScale.Minimum"=w3295, "XScale.Maximum"=w3294) -> ()  [unwired: 2 in, 2 out]
                  }
                }
              }
              frame "PL Intensity (cts)", Default {
              }
            }
          }
          event "Center Wavelength (nm)", "Mono2 Motor Pos", "Mono2 Wavelength (nm)": Value Change {
            n2691 = event-data() -> ("CtlRef"=w3297:refnum<vi>, "NewVal"=w3298:dbl)  [unwired: 1 in, 4 out]
            n2692 = property class="DigNum (strict)"(reference=w3297) -> ("Label.Text"=w3296:string)  [unwired: 1 in, 2 out]
            n2693 = case shown="\"Center Wavelength (nm)\", Default" w3296 {
              tunnel: w3298 -> [w3299 w3347 w3397]
              frame "Mono2 Motor Pos" {
                n2694 = local read "ESP 300 On?"() -> (w3300:bool)
                n2695 = case shown="True" w3300 {
                  tunnel: w3299 -> [_ w3303]
                  frame False {
                  }
                  frame True {
                    n2696 = control-ref of="Mono2 Motor Pos"() -> (w3302:refnum<vi>)
                    n2697 = control-ref of="Mono2 Wavelength (nm)"() -> (w3301:refnum<vi>)
                    n2698 = stacked-sequence {
                      tunnel: w3303 -> [_ w3311 _]
                      tunnel: w3302 -> [w3304 w3309 w3343]
                      tunnel: w3301 -> [w3305 w3308 w3344]
                      frame #0 {
                        # "disable controls when moving"
                        n2699 = property class="DigNum (strict)"(reference=w3305, "DisabledEnum"=T28."Disabled and Grayed Out" ("Disabled")) -> ()  [unwired: 1 in, 2 out]
                        n2700 = property class="DigNum (strict)"(reference=w3304, "DisabledEnum"=T28."Disabled and Grayed Out" ("Disabled")) -> ()  [unwired: 1 in, 2 out]
                      }
                      frame #1 {
                        # "move"
                        n2701 = local read "ESP300 COM Port"() -> (w3310:refnum<visa-resource-name>)
                        n2702 = disable-structure shown="Enabled" {
                          disable-tunnel: w3311 -> [w3319 w3335]
                          disable-tunnel: w3310 -> [w3315 w3336]
                          disable-tunnel: w3309 -> [w3312 w3337]
                          disable-tunnel: w3308 -> [_ w3333]
                          frame Disabled {
                            w3316 = 1 ("Axis")
                            n2703 = call "QMotor On.vi"("Axis"=w3316, "VISA resource name in"=w3315) -> ("error out"=w3322:errorcluster, "Motor On?"=w3324:bool, "VISA resource name out"=w3323:refnum<visa-resource-name>)  [unwired: 7 in]
                            n2704 = case shown="False" w3324 {
                              tunnel: w3316 -> [w3329 _]
                              tunnel: w3323 -> [w3328 w3331]
                              tunnel: w3322 -> [w3327 w3330]
                              tunnel: [w3326 w3331] -> w3321
                              tunnel: [w3325 w3330] -> w3320
                              frame False {
                                n2705 = call "Motor On.vi"("error in (no error)"=w3327, "Axis"=w3329, "VISA resource name in"=w3328) -> ("error out"=w3325:errorcluster, "VISA resource name out"=w3326:refnum<visa-resource-name>)  [unwired: 7 in]
                              }
                              frame True {
                              }
                            }
                            n2706 = call "Move To Position.vi"("error in (no error)"=w3320, "Postion (Unit)"=w3319, "Axis"=w3316, "VISA resource name in"=w3321) -> ("error out"=w3317:errorcluster, "VISA resource name out"=w3318:refnum<visa-resource-name>)  [unwired: 6 in]
                            n2707 = call "Wait For Motion Done.vi"("error in (no error)"=w3317, "Mono2 Motor Pos"=w3312, "Axis"=w3316, "VISA resource name"=w3318) -> ("error out"=w3313:errorcluster, "VISA resource name out"=w3314:refnum<visa-resource-name>)  [unwired: 6 in]
                            n2708 = local write "ESP300 COM Port"(w3314) -> ()
                            n2709 = local write "ESP300 Error"(w3313) -> ()
                          }
                          frame Enabled {
                            n2710 = local read "HR mode"() -> (w3332:u16)
                            n2711 = case shown="0, Default" w3332 {
                              tunnel: w3337 -> [w3342]
                              tunnel: w3336 -> [w3341]
                              tunnel: w3335 -> [w3340]
                              tunnel: w3333 -> [w3339]
                              tunnel: w3332 -> [w3338]
                              frame 0, Default {
                                n2712 = call "subVI_Mono2Go2Posv2.vi"("Mono2 Motor Pos"=w3342, "Mono2 Wavelength (nm)"=w3339, "HR mode"=w3338, "Postion (Unit)"=w3340, "ESP300 COM Port"=w3341) -> ()  [unwired: 2 out]
                              }
                            }
                            n2713 = call "MotorPos2WL.vi"("Mono2 Motor Position"=w3335, "HR mode"=w3332) -> ("Mono2 Center Wavelength (nm)"=w3334:dbl)
                            n2714 = local write "Mono2 Wavelength (nm)"(w3334) -> ()
                          }
                        }
                      }
                      frame #2 {
                        # "re-enable controls when finished moving"
                        n2715 = property class="DigNum (strict)"(reference=w3344, "DisabledEnum"=T28."Enabled" ("Disabled")) -> ()  [unwired: 1 in, 2 out]
                        n2716 = property class="DigNum (strict)"(reference=w3343, "DisabledEnum"=T28."Enabled" ("Disabled")) -> ()  [unwired: 1 in, 2 out]
                      }
                    }
                  }
                }
              }
              frame "Mono2 Wavelength (nm)" {
                n2717 = local read "ESP 300 On?"() -> (w3348:bool)
                n2718 = case shown="True" w3348 {
                  tunnel: w3347 -> [_ w3351]
                  frame False {
                  }
                  frame True {
                    n2719 = control-ref of="Mono2 Motor Pos"() -> (w3350:refnum<vi>)
                    n2720 = control-ref of="Mono2 Wavelength (nm)"() -> (w3349:refnum<vi>)
                    n2721 = stacked-sequence {
                      tunnel: w3351 -> [_ w3359 _]
                      tunnel: w3350 -> [w3355 w3358 w3394]
                      tunnel: w3349 -> [w3352 w3357 w3392]
                      frame #0 {
                        n2722 = property class="DigNum (strict)"(reference=w3355, "DisabledEnum"=T28."Disabled and Grayed Out" ("Disabled")) -> ()  [unwired: 1 in, 2 out]
                        n2723 = property class="DigNum (strict)"(reference=w3352, "DisabledEnum"=T28."Disabled and Grayed Out" ("Disabled")) -> ()  [unwired: 1 in, 2 out]
                      }
                      frame #1 {
                        n2724 = local read "HR mode"() -> (w3356:u16)
                        n2725 = local read "ESP300 COM Port"() -> (w3360:refnum<visa-resource-name>)
                        n2726 = disable-structure shown="Enabled" {
                          disable-tunnel: w3360 -> [w3364 w3385]
                          disable-tunnel: w3358 -> [w3361 w3386]
                          disable-tunnel: w3359 -> [_ w3384]
                          disable-tunnel: w3357 -> [_ w3382]
                          disable-tunnel: w3356 -> [_ w3381]
                          frame Disabled {
                            w3365 = 1 ("Axis")
                            n2727 = call "QMotor On.vi"("Axis"=w3365, "VISA resource name in"=w3364) -> ("error out"=w3371:errorcluster, "Motor On?"=w3373:bool, "VISA resource name out"=w3372:refnum<visa-resource-name>)  [unwired: 7 in]
                            n2728 = case shown="False" w3373 {
                              tunnel: w3365 -> [w3378 _]
                              tunnel: w3372 -> [w3377 w3380]
                              tunnel: w3371 -> [w3376 w3379]
                              tunnel: [w3375 w3380] -> w3370
                              tunnel: [w3374 w3379] -> w3369
                              frame False {
                                n2729 = call "Motor On.vi"("error in (no error)"=w3376, "Axis"=w3378, "VISA resource name in"=w3377) -> ("error out"=w3374:errorcluster, "VISA resource name out"=w3375:refnum<visa-resource-name>)  [unwired: 7 in]
                              }
                              frame True {
                              }
                            }
                            n2730 = call "Move To Position.vi"("error in (no error)"=w3369, "Axis"=w3365, "VISA resource name in"=w3370) -> ("error out"=w3366:errorcluster, "VISA resource name out"=w3367:refnum<visa-resource-name>, "Postion (Unit)"=w3368:dbl)  [unwired: 6 in]
                            n2731 = call "Wait For Motion Done.vi"("error in (no error)"=w3366, "Mono2 Motor Pos"=w3361, "Axis"=w3365, "VISA resource name"=w3367) -> ("error out"=w3362:errorcluster, "VISA resource name out"=w3363:refnum<visa-resource-name>)  [unwired: 6 in]
                            n2732 = local write "ESP300 COM Port"(w3363) -> ()
                            n2733 = local write "ESP300 Error"(w3362) -> ()
                          }
                          frame Enabled {
                            n2734 = call "MotorWL2Pos.vi"("Mono2 Center WL"=w3384, "HR mode"=w3381) -> ("Mono2 Position"=w3383:dbl)
                            n2735 = case shown="0, Default" w3381 {
                              tunnel: w3386 -> [w3391]
                              tunnel: w3385 -> [w3390]
                              tunnel: w3383 -> [w3389]
                              tunnel: w3382 -> [w3388]
                              tunnel: w3381 -> [w3387]
                              frame 0, Default {
                                n2736 = call "subVI_Mono2Go2Posv2.vi"("Mono2 Motor Pos"=w3391, "Mono2 Wavelength (nm)"=w3388, "HR mode"=w3387, "Postion (Unit)"=w3389, "ESP300 COM Port"=w3390) -> ()  [unwired: 2 out]
                              }
                            }
                            n2737 = local write "Mono2 Motor Pos"(w3383) -> ()
                          }
                        }
                      }
                      frame #2 {
                        n2738 = property class="DigNum (strict)"(reference=w3392, "DisabledEnum"=T28."Enabled" ("Disabled")) -> ()  [unwired: 1 in, 2 out]
                        n2739 = property class="DigNum (strict)"(reference=w3394, "DisabledEnum"=T28."Enabled" ("Disabled")) -> ()  [unwired: 1 in, 2 out]
                      }
                    }
                  }
                }
              }
              frame "Center Wavelength (nm)", Default {
                n2740 = local read "LightField On?"() -> (w3396:bool)
                n2741 = case shown="True" w3396 {
                  tunnel: w3397 -> [_ w3398]
                  frame False {
                  }
                  frame True {
                    n2742 = local read "LightField Automation error out"() -> (w3403:errorcluster)
                    n2743 = local read "LightField Automation out"() -> (w3404:refnum<class "LightField Automation.lvclass">)
                    n2744 = call "spec_GetCenterWavelength.vi"("error in (no error)"=w3403, "LightField Automation in"=w3404) -> ("error out"=w3399:errorcluster, "Center Wavelength"=w3402:dbl, "LightField Automation out"=w3400:refnum<class "LightField Automation.lvclass">)  [unwired: 7 in]
                    n2745 = Equal?(x=w3398, y=w3402) -> (x = y?=w3401:bool)
                    n2746 = case shown="False" w3401 {
                      tunnel: w3400 -> [w3407 w3419]
                      tunnel: w3399 -> [w3406 w3418]
                      tunnel: w3398 -> [w3405 _]
                      frame False {
                        n2747 = stacked-sequence {
                          tunnel: w3407 -> [_ w3411 _]
                          tunnel: w3406 -> [_ w3410 _]
                          tunnel: w3405 -> [_ w3409 _]
                          frame #0 {
                            w3408 = T28."Disabled and Grayed Out" ("Disabled")
                            n2748 = property on="Center Wavelength (nm)" class="DigNum (strict)"("DisabledEnum"=w3408) -> ()  [unwired: 2 in, 2 out]
                            n2749 = property on="Grating" class="CmbBox"("DisabledEnum"=w3408) -> ()  [unwired: 2 in, 2 out]
                            n2750 = property on="Exit mirror" class="Ring (strict)"("DisabledEnum"=w3408) -> ()  [unwired: 2 in, 2 out]
                          }
                          frame #1 {
                            n2751 = call "spec_SetCenterWavelength.vi"("error in (no error)"=w3410, "Center Wavelength"=w3409, "LightField Automation in"=w3411) -> ("error out"=w3415:errorcluster, "LightField Automation out"=w3416:refnum<class "LightField Automation.lvclass">)  [unwired: 7 in]
                            n2752 = call "spec_getCalibration.vi"("error in (no error)"=w3415, "LightField Automation in"=w3416) -> ("error out"=w3413:errorcluster, "ColumnCalibration"=w3414:dbl[], "LightField Automation out"=w3412:refnum<class "LightField Automation.lvclass">)  [unwired: 7 in]
                            n2753 = local write "LightField Automation error out"(w3413) -> ()
                            n2754 = local write "LightField Automation out"(w3412) -> ()
                            n2755 = local write "Wavelength calibration"(w3414) -> ()
                          }
                          frame #2 {
                            w3417 = T28."Enabled" ("Disabled")
                            n2756 = property on="Center Wavelength (nm)" class="DigNum (strict)"("DisabledEnum"=w3417) -> ()  [unwired: 2 in, 2 out]
                            n2757 = property on="Grating" class="CmbBox"("DisabledEnum"=w3417) -> ()  [unwired: 2 in, 2 out]
                            n2758 = property on="Exit mirror" class="Ring (strict)"("DisabledEnum"=w3417) -> ()  [unwired: 2 in, 2 out]
                          }
                        }
                      }
                      frame True {
                        n2759 = local write "LightField Automation error out"(w3418) -> ()
                        n2760 = local write "LightField Automation out"(w3419) -> ()
                      }
                    }
                  }
                }
              }
            }
          }
          event "Conv/Energy (eV)", "Conv/Wavelength (nm)", "Conv/Time (s)", "Conv/Wavenumber (m-1)": Value Change {
            n2761 = event-data() -> ("CtlRef"=w3422:refnum<vi>, "NewVal"=w3420:dbl)  [unwired: 1 in, 4 out]
            n2762 = property class="DigNum (strict)"(reference=w3422) -> ("Label.Text"=w3421:string)  [unwired: 1 in, 2 out]
            n2763 = case shown="\"Conv/Energy (eV)\"" w3421 {
              tunnel: w3420 -> [w3430 _ w3443 _]
              frame "Conv/Wavelength (nm)", Default {
                n2764 = Multiply(x=w3430, y=1e-09) -> (x*y=w3428:dbl)
                n2765 = Divide(x=1.0, y=w3428) -> (x/y=w3425:dbl)
                n2766 = Divide(x=w3428, y=299792458.0) -> (x/y=w3427:dbl)
                n2767 = Divide(x=w3425, y=100.0) -> (x/y=w3423:dbl)
                n2768 = Divide(x=1239.842, y=w3430) -> (x/y=w3432:dbl)
                n2769 = local write "Conv/Energy (eV)"(w3432) -> ()
                n2770 = local write "Conv/Wavenumber (m-1)"(w3423) -> ()
                n2771 = local write "Conv/Time (s)"(w3427) -> ()
              }
              frame "Conv/Time (s)" {
              }
              frame "Conv/Energy (eV)" {
                n2772 = Divide(x=1239.842, y=w3443) -> (x/y=w3442:dbl)
                n2773 = Multiply(x=w3442, y=1e-09) -> (x*y=w3439:dbl)
                n2774 = local write "Conv/Wavelength (nm)"(w3442) -> ()
                n2775 = Divide(x=1.0, y=w3439) -> (x/y=w3436:dbl)